vi "IMAQdx_AbsImage_Flea3_v4.7.vi"() -> ()   [LabVIEW 2013] (continued)
ODTpowHLat(DipPowHLat)\t0\tVimaging\t0\t0\t1\t0\t1\t1\t0\tbMOTpow(0.5)\tProbePow\t0\tXshimrMOT\tYshimrMOT\tZshimVar\tODTpowZ(DipPowZ)\tVimaging\t0\t0\tHimaging\t0\t0\t0\t0\t0\t0\t0\t0\t0\t0\t0\t0\t0\t0\trMOTdelta(-(rMOTstirDetI +stirWidthF/2))\tODTpowBlue(0)\tODTpowXY(DipPowCr)\tvarWaveP2\tProbePow2\tAmp688(depumpPow)\trMOTpow3\tODTpowX(DipPowX2)\tfreq\tHeatingAmp\t0\tSine\tDetuning\tsingleFreqDet +20\tDoppCoolDet-DoppCoolSweep\tdopCoolT*1000\tDetuning\tsingleFreqStirDet + 20\tsingleFreqStirDet + SFramp + SFramp2\tloadT*1000\tBlueBN\tBlueLaserProbeBN\tSSteckBN\tShortSteckDDS\tPixisPos(TOF)\tCycle Wait for Move\t0\t0\t0\t0\t0\t0\t0\t0\t0\t0\t0\t0\t0\t0\t0\t0\t0\t0\t0\t0\t0\t0\t0\t0\r\narm DIP FLEA\t\tRamp\t1\tcameraArmT\t0\t0\t0\t0\t0\t0\t0\t0\t0\t0\t0\t0\t0\t0\t0\t0\t0\t0\t0\t0\t0\t0\t0\t0\t0\t1\t1\t0\t0\t0\t1\t0\t0\tplus_zman\tminus_zman\tcompensation\trMOTcurrF\trMOTpow3\tcombAmplitude(combWidthF)\trMOTdelta(-(rMOTbroadDetuningF +combWidthF/2))\tODTpowHLat(DipPowHLat)\t0\tVimaging\t0\t0\t0\t0\t1\t0\t0\tbMOTpow(0.5)\tProbePow\t0\tXshimrMOT\tYshimrMOT\tZshimVar\tODTpowZ(DipPowZ3)\tVimaging\t0\t0\tHimaging\t0\t0\t0\t0\t0\t0\t0\t0\t0\t0\t0\t0\t0\t0\trMOTdelta(-(rMOTstirDetI +stirWidthF/2))\tODTpowBlue(0)\tODTpowXY(DipPowCrTOF)\tvarWaveP1\tProbePow2\tAmp688(depumpPow)\trMOTpow3\tODTpowX(DipPowXTOF)\tfreq\tHeatingAmp\t0\tSine\tDetuning\tsingleFreqDet +20\tDoppCoolDet-DoppCoolSweep\tdopCoolT*1000\tDetuning\tsingleFreqStirDet + 20\tsingleFreqStirDet + SFramp + SFramp2\tloadT*1000\tBlueBN\tBlueLaserProbeBN\tSSteckBN\tShortSteckDDS\tPixisPos(TOF)\tCycle Wait for Move\t0\t0\t0\t0\t0\t0\t0\t0\t0\t0\t0\t0\t0\t0\t0\t0\t0\t0\t0\t0\t0\t0\t0\t0\r\narm BEC FLEA\t\tRamp\t0\tcameraArmT\t1\t1\t1\t1\t1\t1\t0\t0\t0\t0\t0\t0\t0\t0\t0\t0\t0\t0\t0\t0\t0\t0\t0\t0\t0\t1\t1\t0\t0\t0\t1\t0\t0\tplus_zman\tminus_zman\tcompensation\trMOTcurrF\trMOTpow3\tcombAmplitude(combWidthF)\trMOTdelta(-(rMOTbroadDetuningF +combWidthF/2))\tODTpowHLat(DipPowHLat)\t0\tVimaging\t0\t0\t0\t0\t1\t0\t0\tbMOTpow(0.5)\tProbePow\t0\tXshimrMOT\tYshimrMOT\tZshimVar\tODTpowZ(DipPowZ3)\tVimaging\t0\t0\tHimaging\t0\t0\t0\t0\t0\t0\t0\t0\t0\t0\t0\t0\t0\t0\trMOTdelta(-(rMOTstirDetI +stirWidthF/2))\tODTpowBlue(BlueDipPow)\tExpFinal(tEvap1,ODTpowXY(DipPowCr2),ODTpowXY(DipPowCr3),tau)\tvarWaveP1\tProbePow2\tAmp688(depumpPow)\trMOTpow3\tExpFinal(tEvap1,ODTpowX(DipPowX2),ODTpowX(DipPowX3),tau)\tfreq\tHeatingAmp\t0\tSine\tDetuning\tsingleFreqDet +20\tDoppCoolDet-DoppCoolSweep\tdopCoolT*1000\tDetuning\tsingleFreqStirDet + 20\tsingleFreqStirDet + SFramp + SFramp2\tloadT*1000\tBlueBN\tBlueLaserProbeBN\tSSteckBN\tShortSteckDDS\tPixisPos(TOF)\tCycle Wait for Move\t0\t0\t0\t0\t0\t0\t0\t0\t0\t0\t0\t0\t0\t0\t0\t0\t0\t0\t0\t0\t0\t0\t0\t0\r\natom img\t\tRamp\t1\texposureT\t0\t0\t0\t0\t0\t0\t0\t0\t1\t0\t0\t0\t0\t1\t0\t0\t0\t0\t1\t0\t0\t0\t0\t0\t0\t1\t1\t0\t0\t0\t1\t0\t0\tplus_zman\tminus_zman\tcompensation\trMOTcurrF\trMOTpow3\tcombAmplitude(combWidthF)\trMOTdelta(-(rMOTbroadDetuningF +combWidthF/2))\tODTpowHLat(DipPowHLat)\t0\tVimaging\t0\t0\t0\t0\t0\t0\t0\tbMOTpow(0.5)\tProbePow\t0\tXshimrMOT\tYshimrMOT\tZshimVar\tODTpowZ(DipPowZ)\tVimaging\t0\t0\tHimaging\t0\t0\t0\t0\t0\t0\t0\t0\t0\t0\t0\t0\t0\t0\trMOTdelta(-(rMOTstirDetI +stirWidthF/2))\tODTpowBlue(BlueDipPow)\tODTpowXY(DipPowCr)\tvarWaveP1\tProbePow2\tAmp688(depumpPow)\trMOTpow3\tODTpowX(DipPowX)\tfreq\tHeatingAmp\t0\tSine\tDetuning\tsingleFreqDet +20\tDoppCoolDet-DoppCoolSweep\tdopCoolT*1000\tDetuning\tsingleFreqStirDet + 20\tsingleFreqStirDet + SFramp + SFramp2\tloadT*1000\tBlueBN\tBlueLaserProbeBN\tSSteckBN\tShortSteckDDS\tPixisPos(TOF)\tCycle Wait for Move\t0\t0\t0\t0\t0\t0\t0\t0\t0\t0\t0\t0\t0\t0\t0\t0\t0\t0\t0\t0\t0\t0\t0\t0\r\natom img\t\tRamp\t0\t2.8e-3\t0\t0\t0\t0\t0\t0\t0\t0\t0\t1\t0\t0\t0\t0\t0\t0\t0\t0\t0\t0\t0\t0\t0\t0\t0\t1\t1\t0\t0\t0\t1\t1\t0\tplus_zman\tminus_zman\tcompensation\trMOTcurrF\trMOTpow3\tcombAmplitude(combWidthF)\trMOTdelta(-(rMOTbroadDetuningF +combWidthF/2))\tODTpowHLat(DipPowHLat)\t0\tVimaging\t0\t0\t1\t0\t1\t1\t0\tbMOTpow(0.5)\tProbePow\t0\tXshimrMOT\tYshimrMOT\tZshimVar\tODTpowZ(DipPowZ)\tVimaging\t0\t0\tHimaging\t0\t0\t0\t0\t0\t0\t0\t0\t0\t0\t0\t0\t0\t0\trMOTdelta(-(rMOTstirDetI +stirWidthF/2))\tODTpowBlue(0)\tODTpowXY(DipPowCr)\tvarWaveP2\tProbePow2\tAmp688(depumpPow)\trMOTpow3\tODTpowX(DipPowX)\tfreq\tHeatingAmp\t0\tSine\tDetuning\tsingleFreqDet +20\tDoppCoolDet-DoppCoolSweep\tdopCoolT*1000\tDetuning\tsingleFreqStirDet + 20\tsingleFreqStirDet + SFramp + SFramp2\tloadT*1000\tBlueBN\tBlueLaserProbeBN\tSSteckBN\tShortSteckDDS\tPixisPos(TOF)\tCycle Wait for Move\t0\t0\t0\t0\t0\t0\t0\t0\t0\t0\t0\t0\t0\t0\t0\t0\t0\t0\t0\t0\t0\t0\t0\t0\r\ntransmit img\t\tRamp\t1\t.7\t0\t0\t0\t0\t0\t0\t0\t0\t0\t1\t0\t0\t0\t0\t0\t0\t0\t0\t0\t0\t0\t0\t0\t0\t0\t1\t1\t0\t0\t0\t1\t1\t0\tplus_zman\tminus_zman\tcompensation\trMOTcurrF\trMOTpow3\tcombAmplitude(combWidthF)\trMOTdelta(-(rMOTbroadDetuningF +combWidthF/2))\tODTpowHLat(DipPowHLat)\t0\tVimaging\t0\t0\t1\t0\t1\t1\t0\tbMOTpow(0.5)\tProbePow\t0\tXshimrMOT\tYshimrMOT\tZshimVar\tODTpowZ(DipPowZ)\tVimaging\t0\t0\t1\t0\t1\t0\t0\t0\t0\t0\t0\t0\t0\t0\t0\t0\t0\trMOTdelta(-(rMOTstirDetI +stirWidthF/2))\tODTpowBlue(0)\tODTpowXY(DipPowCr)\tvarWaveP2\tProbePow2\tAmp688(depumpPow)\trMOTpow3\tODTpowX(DipPowX)\tfreq\tHeatingAmp\t0\tSine\tDetuning\tsingleFreqDet +20\tDoppCoolDet-DoppCoolSweep\tdopCoolT*1000\tDetuning\tsingleFreqStirDet + 20\tsingleFreqStirDet + SFramp + SFramp2\tloadT*1000\tBlueBN\tBlueLaserProbeBN\tSSteckBN\tShortSteckDDS\tPixisPos(TOF)\tCycle Wait for Move\t0\t0\t0\t0\t0\t0\t0\t0\t0\t0\t0\t0\t0\t0\t0\t0\t0\t0\t0\t0\t0\t0\t0\t0\r\narm PIXIS\t\tRamp\t0\t.007\t0\t0\t0\t0\t0\t0\t0\t0\t0\t1\t1\t0\t0\t0\t1\t1\t0\t0\t0\t0\t0\t0\t0\t0\t0\t1\t1\t0\t0\t0\t1\t1\t0\tplus_zman\tminus_zman\tcompensation\trMOTcurrF\trMOTpow1\tcombAmplitude(combWidthF)\trMOTdelta(-(rMOTbroadDetuningF +combWidthF/2))\tODTpowHLat(DipPowHLat)\t0\tVimaging\t0\t0\t1\t0\t1\t1\t0\tbMOTpow(0.5)\tProbePow\t0\tXshimrMOT\tYshimrMOT\tZshimVar\tODTpowZ(DipPowZ)\tVimaging\t0\t0\t1\t0\t1\t0\t0\t0\t0\t0\t0\t0\t0\t0\t0\t0\t0\trMOTdelta(-(rMOTstirDetI +stirWidthF/2))\tODTpowBlue(0)\tODTpowXY(DipPowCr)\tvarWaveP2\tProbePow2\tAmp688(depumpPow)\trMOTpow1\tODTpowX(DipPowX)\tfreq\tHeatingAmp\t0\tSine\tDetuning\tsingleFreqDet +20\tDoppCoolDet-DoppCoolSweep\tdopCoolT*1000\tDetuning\tsingleFreqStirDet + 20\tsingleFreqStirDet + SFramp + SFramp2\tloadT*1000\tBlueBN\tBlueLaserProbeBN\tSSteckBN\tShortSteckDDS\tPixisPos(TOF)\tCycle Wait for Move\t0\t0\t0\t0\t0\t0\t0\t0\t0\t0\t0\t0\t0\t0\t0\t0\t0\t0\t0\t0\t0\t0\t0\t0\r\narm FLEA\t\tRamp\t1\tcameraArmT\t0\t0\t0\t0\t0\t0\t0\t0\t0\t1\t1\t0\t0\t0\t1\t1\t0\t0\t0\t0\t0\t0\t0\t0\t0\t1\t1\t0\t0\t0\t1\t0\t0\tplus_zman\tminus_zman\tcompensation\trMOTcurrF\trMOTpow1\tcombAmplitude(combWidthF)\trMOTdelta(-(rMOTbroadDetuningF +combWidthF/2))\tODTpowHLat(DipPowHLat)\t0\tVimaging\t0\t0\t0\t0\t1\t0\t0\tbMOTpow(0.5)\tProbePow\t0\tXshimrMOT\tYshimrMOT\tZshimVar\tODTpowZ(DipPowZ)\tVimaging\t0\t0\t0\t0\t1\t0\t0\t0\t0\t0\t0\t0\t0\t0\t0\t0\t0\trMOTdelta(-(rMOTstirDetI +stirWidthF/2))\tODTpowBlue(0)\tODTpowXY(DipPowCr)\tvarWaveP2\tProbePow2\tAmp688(depumpPow)\trMOTpow1\tODTpowX(DipPowX)\tfreq\tHeatingAmp\t0\tSine\tDetuning\tsingleFreqDet +20\tDoppCoolDet-DoppCoolSweep\tdopCoolT*1000\tDetuning\tsingleFreqStirDet + 20\tsingleFreqStirDet + SFramp + SFramp2\tloadT*1000\tBlueBN\tBlueLaserProbeBN\tSSteckBN\tShortSteckDDS\tPixisPos(TOF)\tCycle Wait for Move\t0\t0\t0\t0\t0\t0\t0\t0\t0\t0\t0\t0\t0\t0\t0\t0\t0\t0\t0\t0\t0\t0\t0\t0\r\nprobe img\t\tRamp\t1\texposureT\t0\t0\t0\t0\t0\t0\t0\t0\t1\t1\t1\t0\t0\t1\t1\t1\t0\t0\t0\t0\t0\t0\t0\t0\t0\t1\t1\t0\t0\t0\t1\t0\t0\tplus_zman\tminus_zman\tcompensation\trMOTcurrF\trMOTpow1\tcombAmplitude(combWidthF)\trMOTdelta(-(rMOTbroadDetuningF +combWidthF/2))\tODTpowHLat(DipPowHLat)\t0\tVimaging\t0\t0\t0\t0\t0\t0\t0\tbMOTpow(0.5)\tProbePow\t0\tXshimrMOT\tYshimrMOT\tZshimVar\tODTpowZ(DipPowZ)\tVimaging\t0\t0\t0\t0\t1\t0\t0\t0\t0\t0\t0\t0\t0\t0\t0\t0\t0\trMOTdelta(-(rMOTstirDetI +stirWidthF/2))\tODTpowBlue(0)\tODTpowXY(DipPowCr)\tvarWaveP2\tProbePow2\tAmp688(depumpPow)\trMOTpow1\tODTpowX(DipPowX)\tfreq\tHeatingAmp\t0\tSine\tDetuning\tsingleFreqDet +20\tDoppCoolDet-DoppCoolSweep\tdopCoolT*1000\tDetuning\tsingleFreqStirDet + 20\tsingleFreqStirDet + SFramp + SFramp2\tloadT*1000\tBlueBN\tBlueLaserProbeBN\tSSteckBN\tShortSteckDDS\tPixisPos(TOF)\tCycle Wait for Move\t0\t0\t0\t0\t0\t0\t0\t0\t0\t0\t0\t0\t0\t0\t0\t0\t0\t0\t0\t0\t0\t0\t0\t0\r\nprobe img\t\tRamp\t0\t2.8e-3\t0\t0\t0\t0\t0\t0\t0\t0\t0\t1\t1\t0\t0\t0\t1\t1\t0\t0\t0\t0\t0\t0\t0\t0\t0\t1\t1\t0\t0\t0\t1\t1\t0\tplus_zman\tminus_zman\tcompensation\trMOTcurrF\trMOTpow1\tcombAmplitude(combWidthF)\trMOTdelta(-(rMOTbroadDetuningF +combWidthF/2))\tODTpowHLat(DipPowHLat)\t0\tVimaging\t0\t0\t1\t0\t1\t1\t0\tbMOTpow(0.5)\tProbePow\t0\tXshimrMOT\tYshimrMOT\tZshimVar\tODTpowZ(DipPowZ)\tVimaging\t0\t0\t0\t0\t1\t0\t0\t0\t0\t0\t0\t0\t0\t0\t0\t0\t0\trMOTdelta(-(rMOTstirDetI +stirWidthF/2))\tODTpowBlue(0)\tODTpowXY(DipPowCr)\tvarWaveP2\tProbePow2\tAmp688(depumpPow)\trMOTpow1\tODTpowX(DipPowX)\tfreq\tHeatingAmp\t0\tSine\tDetuning\tsingleFreqDet +20\tDoppCoolDet-DoppCoolSweep\tdopCoolT*1000\tDetuning\tsingleFreqStirDet + 20\tsingleFreqStirDet + SFramp + SFramp2\tloadT*1000\tBlueBN\tBlueLaserProbeBN\tSSteckBN\tShortSteckDDS\tPixisPos(TOF)\tCycle Wait for Move\t0\t0\t0\t0\t0\t0\t0\t0\t0\t0\t0\t0\t0\t0\t0\t0\t0\t0\t0\t0\t0\t0\t0\t0\r\ntransmit img\t\tRamp\t1\t.600\t0\t0\t0\t0\t0\t0\t0\t0\t0\t1\t1\t0\t0\t0\t1\t1\t0\t0\t0\t0\t0\t0\t0\t0\t0\t1\t1\t0\t0\t0\t1\t1\t0\tplus_zman\tminus_zman\tcompensation\trMOTcurrF\trMOTpow1\tcombAmplitude(combWidthF)\trMOTdelta(-(rMOTbroadDetuningF +combWidthF/2))\tODTpowHLat(DipPowHLat)\t0\tVimaging\t0\t0\t1\t0\t1\t1\t0\tbMOTpow(0.5)\tProbePow\t0\tXshimrMOT\tYshimrMOT\tZshimVar\tODTpowZ(DipPowZ)\tVimaging\t0\t0\t0\t0\t1\t0\t0\t0\t0\t0\t0\t0\t0\t0\t0\t0\t0\trMOTdelta(-(rMOTstirDetI +stirWidthF/2))\tODTpowBlue(0)\tODTpowXY(DipPowCr)\tvarWaveP2\tProbePow2\tAmp688(depumpPow)\trMOTpow1\tODTpowX(DipPowX)\tfreq\tHeatingAmp\t0\tSine\tDetuning\tsingleFreqDet +20\tDoppCoolDet-DoppCoolSweep\tdopCoolT*1000\tDetuning\tsingleFreqStirDet + 20\tsingleFreqStirDet + SFramp + SFramp2\tloadT*1000\tBlueBN\tBlueLaserProbeBN\tSSteckBN\tShortSteckDDS\tPixisPos(TOF)\tCycle Wait for Move\t0\t0\t0\t0\t0\t0\t0\t0\t0\t0\t0\t0\t0\t0\t0\t0\t0\t0\t0\t0\t0\t0\t0\t0\r\ntransmit img\t\tRamp\t1\t.025\t0\t0\t0\t0\t0\t0\t0\t0\t0\t1\t1\t0\t0\t0\t1\t1\t0\t0\t0\t0\t0\t0\t0\t0\t0\t1\t1\t0\t0\t0\t1\t1\t0\tplus_zman\tminus_zman\tcompensation\trMOTcurrF\trMOTpow1\tcombAmplitude(combWidthF)\trMOTdelta(-(rMOTbroadDetuningF +combWidthF/2))\tODTpowHLat(DipPowHLat2)\t0\tVimaging\t0\t0\t1\t0\t1\t1\t0\tbMOTpow(0.5)\tProbePow\t0\tXshimrMOT\tYshimrMOT\tZshimVar\tODTpowZ(DipPowZ)\tVimaging\t0\t0\t0\t0\t1\t0\t0\t0\t0\t0\t0\t0\t0\t0\t0\t0\t0\trMOTdelta(-(rMOTstirDetI +stirWidthF/2))\tODTpowBlue(.05)\tODTpowXY(DipPowCr)\tvarWaveP2\tProbePow2\tAmp688(depumpPow)\trMOTpow1\tODTpowX(DipPowX)\tfreq\tHeatingAmp\t0\tSine\tDetuning\tsingleFreqDet +20\tDoppCoolDet-DoppCoolSweep\tdopCoolT*1000\tDetuning\tsingleFreqStirDet + 20\tsingleFreqStirDet + SFramp + SFramp2\tloadT*1000\tBlueBN\tBlueLaserProbeBN\tSSteckBN\tShortSteckDDS\tPixisPos(TOF)\tCycle Wait for Move\t0\t0\t0\t0\t0\t0\t0\t0\t0\t0\t0\t0\t0\t0\t0\t0\t0\t0\t0\t0\t0\t0\t0\t0\r\narm PIXIS\t\tRamp\t0\t.007\t0\t0\t0\t0\t0\t0\t0\t0\t0\t1\t1\t0\t0\t0\t1\t1\t0\t0\t0\t0\t0\t0\t0\t0\t0\t1\t1\t0\t0\t0\t1\t0\t0\tplus_zman\tminus_zman\tcompensation\trMOTcurrF\trMOTpow1\tcombAmplitude(combWidthF)\trMOTdelta(-(rMOTbroadDetuningF +combWidthF/2))\tODTpowHLat(DipPowHLat2)\t0\tVimaging\t0\t0\t0\t0\t1\t1\t0\tbMOTpow(0.5)\tProbePow\t0\tXshimrMOT\tYshimrMOT\tZshimVar\tODTpowZ(DipPowZ)\tVimaging\t0\t0\t0\t0\t1\t0\t0\t0\t0\t0\t0\t0\t0\t0\t0\t0\t0\trMOTdelta(-(rMOTstirDetI +stirWidthF/2))\tODTpowBlue(0)\tODTpowXY(DipPowCr)\tvarWaveP2\tProbePow2\tAmp688(depumpPow)\trMOTpow1\tODTpowX(DipPowX)\tfreq\tHeatingAmp\t0\tSine\tDetuning\tsingleFreqDet +20\tDoppCoolDet-DoppCoolSweep\tdopCoolT*1000\tDetuning\tsingleFreqStirDet + 20\tsingleFreqStirDet + SFramp + SFramp2\tloadT*1000\tBlueBN\tBlueLaserProbeBN\tSSteckBN\tShortSteckDDS\tPixisPos(TOF)\tCycle Wait for Move\t0\t0\t0\t0\t0\t0\t0\t0\t0\t0\t0\t0\t0\t0\t0\t0\t0\t0\t0\t0\t0\t0\t0\t0\r\narm FLEA\t\tRamp\t1\tcameraArmT\t0\t0\t0\t0\t0\t0\t0\t0\t0\t1\t1\t0\t0\t0\t1\t1\t0\t0\t0\t0\t0\t0\t0\t0\t0\t1\t1\t0\t0\t0\t1\t0\t0\tplus_zman\tminus_zman\tcompensation\trMOTcurrF\trMOTpow1\tcombAmplitude(combWidthF)\trMOTdelta(-(rMOTbroadDetuningF +combWidthF/2))\tODTpowHLat(DipPowHLat2)\t0\tVimaging\t0\t0\t0\t0\t1\t0\t0\tbMOTpow(0.5)\tProbePow\t0\tXshimrMOT\tYshimrMOT\tZshimVar\tODTpowZ(DipPowZ)\tVimaging\t0\t0\t0\t0\t1\t0\t0\t0\t0\t0\t0\t0\t0\t0\t0\t0\t0\trMOTdelta(-(rMOTstirDetI +stirWidthF/2))\tODTpowBlue(.05)\tODTpowXY(DipPowCr)\tvarWaveP2\tProbePow2\tAmp688(depumpPow)\trMOTpow1\tODTpowX(DipPowX)\tfreq\tHeatingAmp\t0\tSine\tDetuning\tsingleFreqDet +20\tDoppCoolDet-DoppCoolSweep\tdopCoolT*1000\tDetuning\tsingleFreqStirDet + 20\tsingleFreqStirDet + SFramp + SFramp2\tloadT*1000\tBlueBN\tBlueLaserProbeBN\tSSteckBN\tShortSteckDDS\tPixisPos(TOF)\tCycle Wait for Move\t0\t0\t0\t0\t0\t0\t0\t0\t0\t0\t0\t0\t0\t0\t0\t0\t0\t0\t0\t0\t0\t0\t0\t0\r\nbg img\t\tRamp\t1\texposureT\t0\t0\t0\t0\t0\t0\t0\t0\t0\t1\t1\t0\t0\t0\t1\t1\t0\t0\t0\t0\t0\t0\t0\t0\t0\t1\t1\t0\t0\t0\t1\t0\t0\tplus_zman\tminus_zman\tcompensation\trMOTcurrF\trMOTpow1\tcombAmplitude(combWidthF)\trMOTdelta(-(rMOTbroadDetuningF +combWidthF/2))\tODTpowHLat(DipPowHLat2)\t0\tVimaging\t0\t0\t0\t0\t0\t0\t0\tbMOTpow(0.5)\tProbePow\t0\tXshimrMOT\tYshimrMOT\tZshimVar\tODTpowZ(DipPowZ)\tVimaging\t0\t0\t0\t0\t1\t0\t0\t0\t0\t0\t0\t0\t0\t0\t0\t0\t0\trMOTdelta(-(rMOTstirDetI +stirWidthF/2))\tODTpowBlue(.05)\tODTpowXY(DipPowCr)\tvarWaveP2\tProbePow2\tAmp688(depumpPow)\trMOTpow1\tODTpowX(DipPowX)\tfreq\tHeatingAmp\t0\tSine\tDetuning\tsingleFreqDet +20\tDoppCoolDet-DoppCoolSweep\tdopCoolT*1000\tDetuning\tsingleFreqStirDet + 20\tsingleFreqStirDet + SFramp + SFramp2\tloadT*1000\tBlueBN\tBlueLaserProbeBN\tSSteckBN\tShortSteckDDS\tPixisPos(TOF)\tCycle Wait for Move\t0\t0\t0\t0\t0\t0\t0\t0\t0\t0\t0\t0\t0\t0\t0\t0\t0\t0\t0\t0\t0\t0\t0\t0\r\nbg img\t\tRamp\t0\t1e-4\t0\t0\t0\t0\t0\t0\t0\t0\t0\t1\t1\t0\t0\t0\t1\t1\t0\t0\t0\t0\t0\t0\t0\t0\t0\t1\t1\t0\t0\t0\t1\t1\t0\tplus_zman\tminus_zman\tcompensation\trMOTcurrF\trMOTpow1\tcombAmplitude(combWidthF)\trMOTdelta(-(rMOTbroadDetuningF +combWidthF/2))\tODTpowHLat(DipPowHLat)\t0\tVimaging\t0\t0\t1\t0\t1\t1\t0\tbMOTpow(0.5)\tProbePow\t0\tXshimrMOT\tYshimrMOT\tZshimVar\tODTpowZ(DipPowZ)\tVimaging\t0\t0\t0\t0\t1\t0\t0\t0\t0\t0\t0\t0\t0\t0\t0\t0\t0\trMOTdelta(-(rMOTstirDetI +stirWidthF/2))\tODTpowBlue(0)\tODTpowXY(DipPowCr)\tvarWaveP2\tProbePow2\tAmp688(depumpPow)\trMOTpow1\tODTpowX(DipPowX)\tfreq\tHeatingAmp\t0\tSine\tDetuning\tsingleFreqDet +20\tDoppCoolDet-DoppCoolSweep\tdopCoolT*1000\tDetuning\tsingleFreqStirDet + 20\tsingleFreqStirDet + SFramp + SFramp2\tloadT*1000\tBlueBN\tBlueLaserProbeBN\tSSteckBN\tShortSteckDDS\tPixisPos(TOF)\tCycle Wait for Move\t0\t0\t0\t0\t0\t0\t0\t0\t0\t0\t0\t0\t0\t0\t0\t0\t0\t0\t0\t0\t0\t0\t0\t0\r\ntransmit img\t\tRamp\t1\t.625\t0\t0\t0\t0\t0\t0\t0\t1\t0\t1\t1\t0\t0\t0\t1\t1\t0\t0\t0\t0\t0\t0\t0\t0\t0\t1\t1\t0\t0\t0\t1\t1\t0\tplus_zman\tminus_zman\tcompensation\trMOTcurrF\trMOTpow1\tcombAmplitude(combWidthF)\trMOTdelta(-(rMOTbroadDetuningF +combWidthF/2))\tODTpowHLat(DipPowHLat)\t0\tVimaging\t0\t0\t1\t0\t1\t1\t0\tbMOTpow(0.5)\tProbePow\t0\tXshimrMOT\tYshimrMOT\tZshimVar\tODTpowZ(DipPowZ)\tVimaging\t0\t0\t0\t0\t1\t0\t0\t0\t0\t0\t0\t0\t0\t0\t0\t0\t0\trMOTdelta(-(rMOTstirDetI +stirWidthF/2))\tODTpowBlue(0)\tODTpowXY(DipPowCr)\tvarWaveP2\tProbePow2\tAmp688(depumpPow)\trMOTpow1\tODTpowX(DipPowX)\tfreq\tHeatingAmp\t0\tSine\tDetuning\tsingleFreqDet +20\tDoppCoolDet-DoppCoolSweep\tdopCoolT*1000\tDetuning\tsingleFreqStirDet + 20\tsingleFreqStirDet + SFramp + SFramp2\tloadT*1000\tBlueBN\tBlueLaserProbeBN\tSSteckBN\tShortSteckDDS\tPixisPos(TOF)\tCycle Wait for Move\t0\t0\t0\t0\t0\t0\t0\t0\t0\t0\t0\t0\t0\t0\t0\t0\t0\t0\t0\t0\t0\t0\t0\t0\r\nalignment\t\tRamp\t1\t.1\t1\t1\t1\t1\t1\t1\t1\t0\t1\t0\t1\t0\t1\t1\t1\t1\t0\t0\t0\t0\t0\t0\t0\t0\t1m\t1\t1\t0\t1\t0\t0\t1\t1\tplus_zman\tminus_zman\tcompensation\tMOTcurrent\trMOTpow1\tcombAmplitude(combWidthI)\trMOTdelta(-(rMOTbroadDetuningI +combWidthI/2))\tODTpowHLat(DipPowHLat2)\t1\t0\t1\t1\t1\t1\t1\t1\t0\tbMOTpow(MOTPow)\tProbePow\t0\tXshim\tYshim\tZshim\tODTpowZ(DipPowZ3)\t0\t1\t1\t0\t1\t1\t0\t1\t0\t0\t0\t0\t0\t0\t0\t0\t0\t0\trMOTdelta(-(rMOTstirDetI +stirWidthI/2))\tODTpowBlue(0.05)\tExpFinal(tEvap1,ODTpowXY(DipPowCr2),ODTpowXY(DipPowCr3),tau)\tvarWaveP2\tProbePow2\tAmp688(depumpPow)\trMOTpow3\tExpFinal(tEvap1,ODTpowX(DipPowX2),ODTpowX(DipPowX3),tau)\tfreq\tHeatingAmp\t0\tSine\tDetuning\tsingleFreqDet +20\tDoppCoolDet-DoppCoolSweep\tdopCoolT*1000\tDetuning\tsingleFreqStirDet + 20\tsingleFreqStirDet + SFramp + SFramp2\tloadT*1000\tBlueBN\tBlueLaserBeatnote\tSSteckBN\tShortSteckDDS\tPixisPos(TOF)\tCycle Wait for Move\t0\t0\t0\t0\t0\t0\t0\t0\t0\t0\t0\t0\t0\t0\t0\t0\t0\t0\t0\t0\t0\t0\t0\t0\r\n\r\n\r\n"
  in  "Flea Wave Name":string="Test_Img"
  in  "Save files to archive?":bool
  out "Timeout":bool
  out "Trigger Overrun":bool
  in  "Source of File Data":refnum<k21>="\\\\Control\\VariableLibrary\\Instruction String"
  in  "Timeout (ms)":u32=20000
  in  "Gain":dbl
  in  "Shutter speed":dbl=30000.0
  in  "PIXIS Magnification":dbl=5.48
  in  "PIXIS Image direction":enum16{"XY", "XZ"}(ring)
  in  "PIXIS Imaging technique":enum16{"Absorption", "Fluorescence", "RawImage"}(ring)
  in  "SPE File Path":path=path "C:/Users/Lab/Documents/LightField/LabviewTemp.spe"
  in  "Send PIXIS data to Igor?":bool
  in  "PIXIS File Parameters":T1={"Data Root"=path "I:/Data", "Index"=3939, "Instrument"="PIXIS"} {"Index" format="%04d"}
  in  "Source of Wavemeter Data":refnum<k21>="\\\\WS7PC\\VariableLibrary\\Frequency"
  in  "Accept wavelength from remote system":bool=TRUE
  in  "Flea Raw image to view":u16(ring) items=["Clear", "Absorbtion", "Probe", "Background"]
  in  "Update Graphics":bool=TRUE
  out "Flea Raw Image":u16[][](graph)
  out "Flea Processed Image":sgl[][](graph)
  out "PIXIS Processed Image":sgl[][](graph)
  out "PIXIS Raw Image":u16[][](graph)
  in  "PIXIS Raw image to view":u16(ring)=1 items=["Clear", "Absorbtion", "Probe", "Background"]
  out "Camera Error":errorcluster
  out "DDE Error":errorcluster={"status"=TRUE, "code"=14012, "source"="DDE Execute: DMLERR_NOTPROCESSED"}
  out "Status Array":T4(array[cluster])=[{"AcquisitionInProgress"=FALSE, "BufferCount"=0, "LastBufferNumber"=4294967292, "LostBufferCount"=0}, {"AcquisitionInProgress"=TRUE, "BufferCount"=0, "LastBufferNumber"=4294967292, "LostBufferCount"=0}, {"AcquisitionInProgress"=TRUE, "BufferCount"=0, "LastBufferNumber"=4294967292, "LostBufferCount"=0}, {"AcquisitionInProgress"=TRUE, "BufferCount"=1, "LastBufferNumber"=0, "LostBufferCount"=0}, {"AcquisitionInProgress"=TRUE, "BufferCount"=2, "LastBufferNumber"=1, "LostBufferCount"=0}, {"AcquisitionInProgress"=TRUE, "BufferCount"=3, "LastBufferNumber"=2, "LostBufferCount"=0}, {"AcquisitionInProgress"=TRUE, "BufferCount"=4, "LastBufferNumber"=3, "LostBufferCount"=0}]
  in  "SPE Load Error In":errorcluster
  out "DataBlock Info":T5={"frame count"=4, "frame size"=2097152, "frame stride"=2097152, "N ROI"=1, "ROI widths"=[1024], "ROI heights"=[1024], "ROI sizes"=[2097152], "ROI strides"=[2097152]}
  out "DS Error":errorcluster
  out "XML Parse Errors":string
  out "Data Array Size":i32=1
  out "SPE Load Error Out":errorcluster
  out "Flea Path":path=path "I:/Data/FL3_32S2Mtemp.ibw"
  out "PIXIS Path":path=path "I:/Data/PIXIStemp.ibw"
  out "PIXIS Images":u16[][][](array[numeric])
  out "Flea Images":u16[][][](array[numeric])
  out "Buffer Number":u32=3
  out "Flea Frames":i32=3
  out "Flea Loop":i32=31
  # "Image Acquisition v4.6 (FOR USB3 CAMERAS ONLY!!!)"
  # "Experimental Parameters"
  # "These are only get set on 1st run.\nUse a Gain of 0, Shutter Speed not used"
  # "In both techniques 3 images\nare aquired, but in Fluorescense\nthe 3rd is discarded"
  # "Sr: .663  is XZ a\n     .898 is XZ b\n      5.48 is XY"
  # "Obsolete: (now done with network variables)\nWhen paramaters are accepted from a remote system a DataSockets server\nmust be running on this machine (in start menu in National Instruments folder)"
  # "Camera configuration"
  # "File configuration"
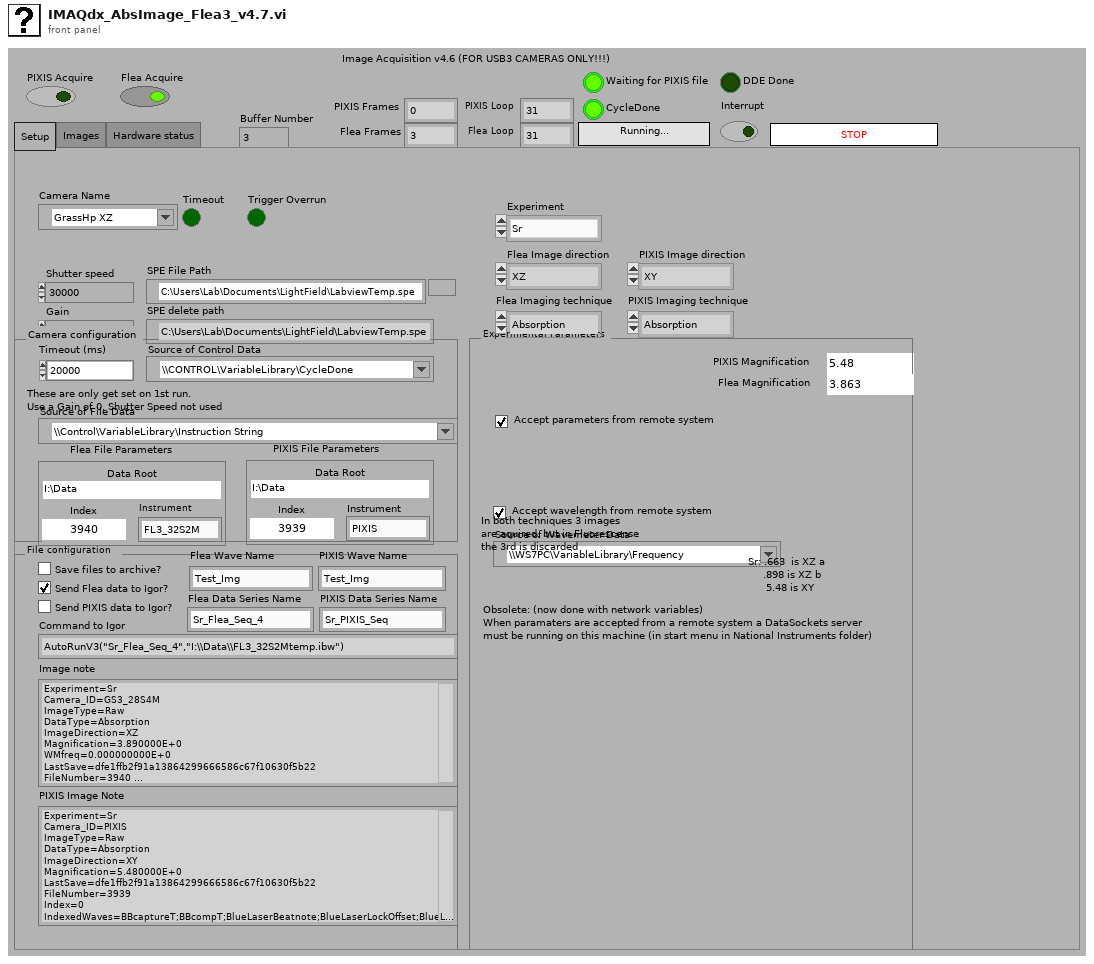
[diagram p1: front panel]
types:
  T1 = typedef "FileName_Cluster.ctl" = cluster{"Data Root":path, "Index":u32, "Instrument":string}
  T2 = typedef "IMAQdx.ctl" = refnum<k21>
  T3 = enum16{"Rubidium I", "Rubidium II", "RbLi", "RbYb", "Sr"}
  T4 = cluster{"AcquisitionInProgress":bool, "BufferCount":u32, "LastBufferNumber":u32, "LostBufferCount":u32}[]
  T5 = cluster{"frame count":i64, "frame size":i64, "frame stride":i64, "N ROI":i64, "ROI widths":i64[], "ROI heights":i64[], "ROI sizes":i64[], "ROI strides":i64[]}
  T6 = typedef "NI_Vision_Acquisition_Software.lvlib/IMAQdx Acquisition Mode.ctl" = enum32{"One Shot", "Continuous"}
  T7 = typedef "Image Type" = u32
  T8 = typedef "IMAQ Image.ctl" = refnum<image>
  T9 = cluster{"AcquisitionInProgress":bool, "BufferCount":u32, "LastBufferNumber":u32, "LostBufferCount":u32}
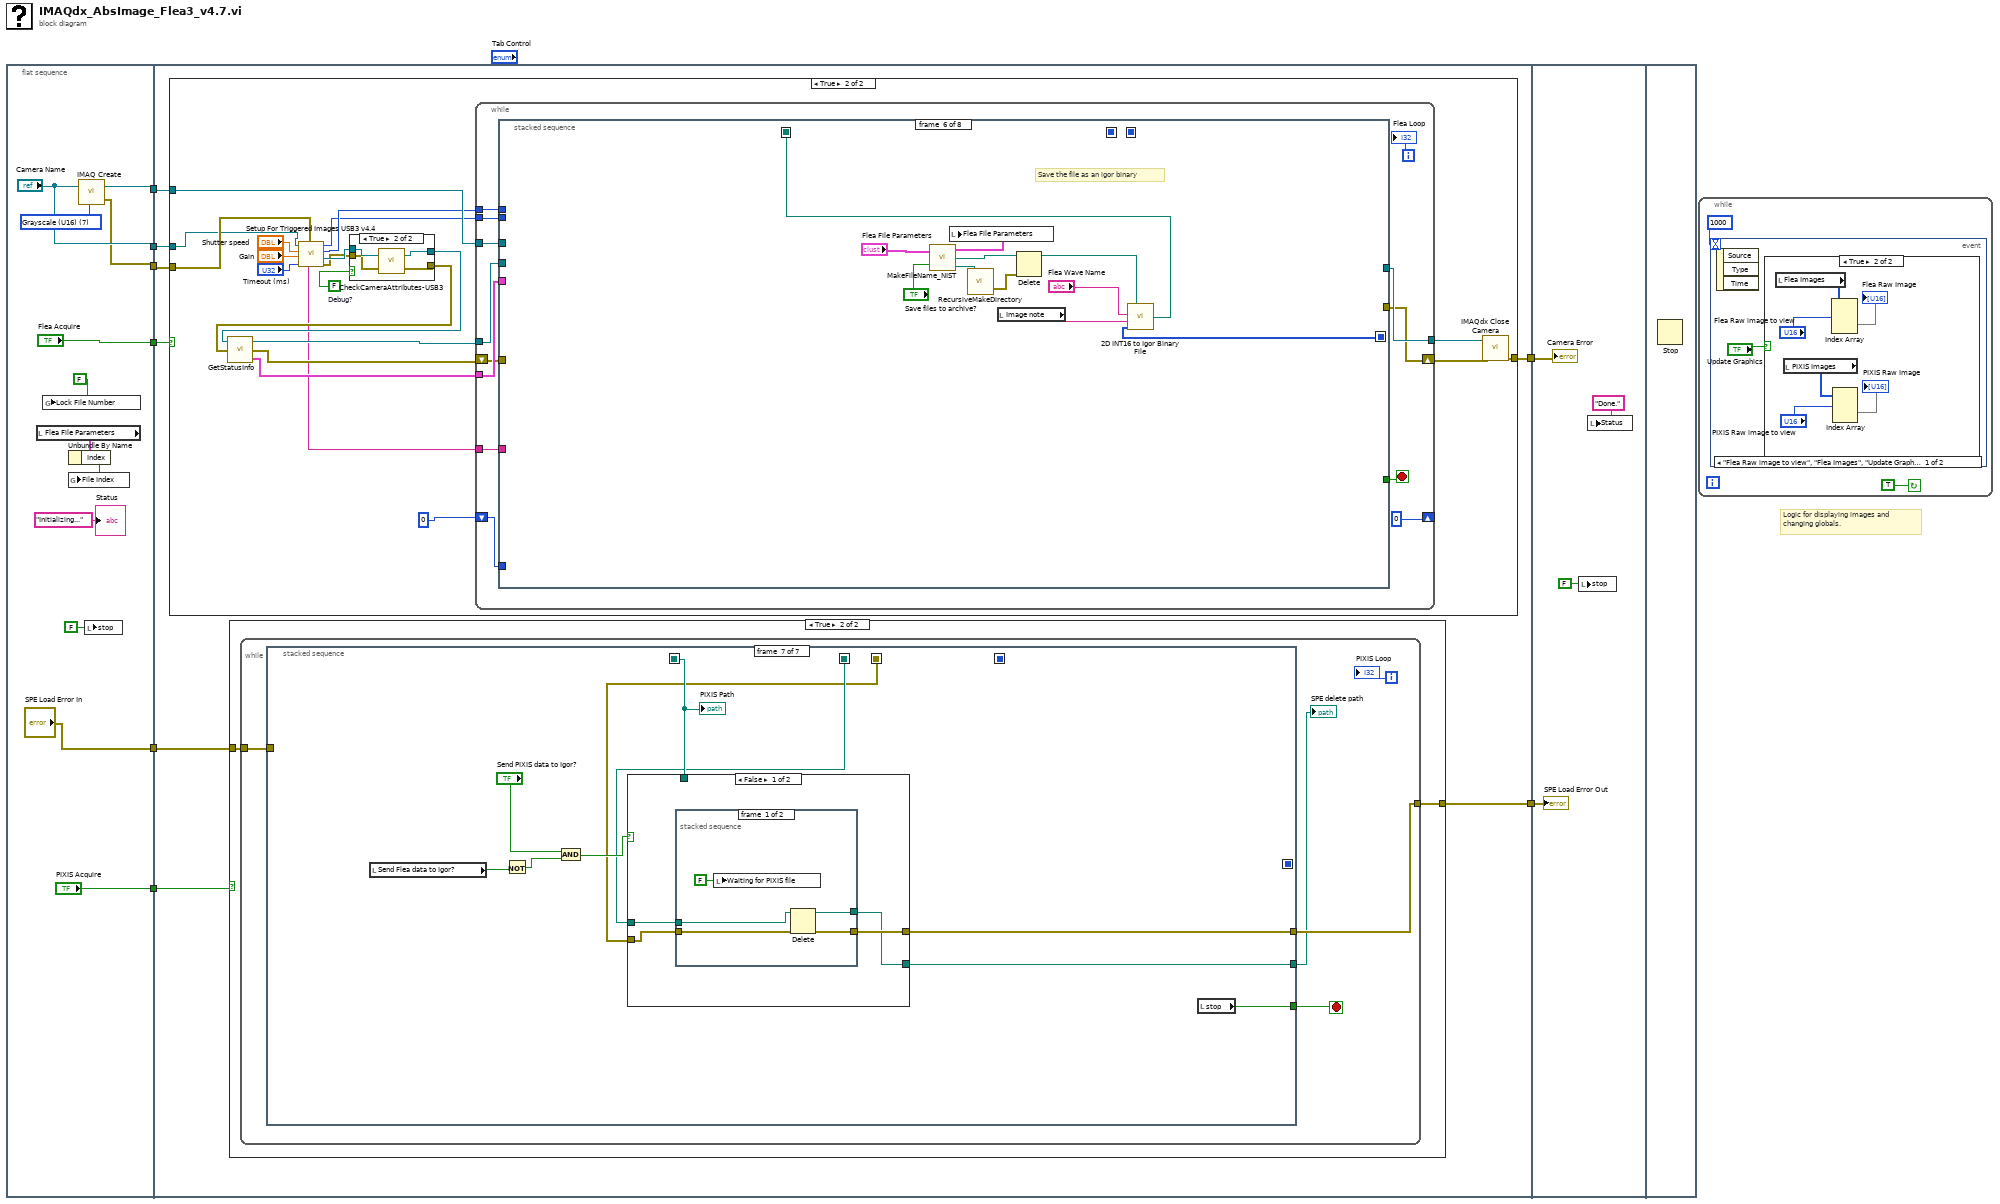
[diagram p0: block diagram]
diagram:
  # "Logic for displaying images and\nchanging globals."
  n1 = flat-sequence {
    tunnel: [w16] -> w8
    tunnel: ["Camera Name"] -> w7
    tunnel: [w14] -> w6
    tunnel: ["SPE Load Error In"] -> w5
    tunnel: ["PIXIS Acquire"] -> w3
    tunnel: ["Flea Acquire"] -> w1
    tunnel: w7 -> [w28]
    tunnel: w8 -> [w26]
    tunnel: w6 -> [w27]
    tunnel: w5 -> [w25]
    tunnel: [w24] -> w4
    tunnel: w3 -> [w23]
    tunnel: [w22] -> w2
    tunnel: w1 -> [w21]
    tunnel: w4 -> [w473]
    tunnel: w2 -> [w472]
    frame #0 {
      w13 = T7 7 items=["Grayscale (U8)", "Grayscale (I16)", "Grayscale (SGL)", "Complex (CSG)", "RGB (U32)", "HSL (U32)", "RGB (U64)", "Grayscale (U16)"] ("Image Type")
      n2 = local read "Flea File Parameters"() -> (w17:T1)
      n3 = global write "FileInfo_Global.vi" "Lock File Number"(FALSE) -> ()
      n4 = Unbundle By Name(w17) -> ("Index"=w18:u32)
      n5 = global write "FileInfo_Global.vi" "File Index"(w18) -> ()
      n6 = call "IMAQ Create"("Image Name"="Camera Name", "Image Type"=w13) -> ("New Image"=w16:T8, "error out"=w14:errorcluster)  [unwired: 2 in, 1 out]
      n7 = local write "stop"(FALSE ("stop")) -> ()
      "Status" <- "Initializing..."
    }
    frame #1 {
      n8 = case shown="True" w21 {
        tunnel: w28 -> [_ w34]
        tunnel: w27 -> [w29 w35]
        tunnel: w26 -> [_ w47]
        tunnel: [w29 w44] -> w22
        frame False {
        }
        frame True {
          w50 = FALSE  # Debug?
          n9 = call "Setup For Triggered Images USB3 v4.4.vi"("error in"=w35, "Timeout"="Timeout (ms)", "Gain"="Gain", "Shutter speed"="Shutter speed", "Camera Name"=w34) -> ("Error out"=w38:errorcluster, "Session Out"=w39:T2, "Height"=w37:u32, "Width"=w36:u32, "DeviceID"=w30:string)
          n10 = case shown="True" w50 {
            tunnel: [w51 w55] -> w49
            tunnel: [w52 w54] -> w48
            tunnel: w39 -> [w51 w56]
            tunnel: w38 -> [w52 w53]
            frame False {
            }
            frame True {
              n11 = call "CheckCameraAttributes-USB3.vi"("error in"=w53, "Camera Name"=w56) -> ("error out"=w54:errorcluster, "Session Out"=w55:T2)
            }
          }
          n12 = call "GetStatusInfo.vi"("error in"=w48, "Camera In"=w49) -> ("Status Info"=w46:T9, "error out"=w43:errorcluster, "Camera Out"=w42:T2)  [unwired: 1 in]
          n13 = while {
            tunnel: w42 -> [w67]
            tunnel: w47 -> [w66]
            tunnel: w37 -> [w65]
            tunnel: w36 -> [w64]
            tunnel: w46 -> [w63]
            tunnel: [w62] -> w41
            shift-right: [0] -> _
            shift-left: 0 -> [w61]
            shift-right: [w58] -> w40
            shift-left: w43 -> [w59]
            tunnel: w30 -> [w57]
            i -> [w69]
            stop <- w68 stop-if-true
            n14 = stacked-sequence {
              seq-local: [_ _ _ w184 _ _ _ _] -> [_ _ _ _ _ w258 _ _]
              seq-local: [_ _ _ _ _ w254 _ _] -> [_ _ _ _ _ _ _ w268]
              seq-local: [_ w89 _ _ _ _ _ _] -> [_ _ w158 _ _ _ _ _]
              seq-local: [_ _ w157 _ _ _ _ _] -> [_ _ _ w175 _ _ _ _]
              tunnel: [_ _ _ _ _ _ _ "stop"] -> w68
              tunnel: w67 -> [_ w81 _ _ _ _ _ _]
              tunnel: w66 -> [_ w97 _ _ _ _ _ _]
              tunnel: w65 -> [_ w96 _ _ _ _ _ _]
              tunnel: w64 -> [_ w95 _ _ _ _ _ _]
              tunnel: w63 -> [_ w93 _ _ _ _ _ _]
              tunnel: [_ w76 _ _ _ _ _ _] -> w62
              tunnel: [_ w75 _ _ _ _ _ _] -> w58
              tunnel: w61 -> [_ w92 _ _ _ _ _ _]
              tunnel: w59 -> [_ w84 _ _ _ _ _ _]
              tunnel: w57 -> [_ _ _ _ w205 _ _ _]
              frame #0 {
                n15 = local read "Send Flea data to Igor?"() -> (w70:bool)
                n16 = local write "Flea Frames"(0) -> ()
                n17 = local write "Status"("Running...") -> ()
                n18 = case shown="False" w70 {
                  frame False {
                    n19 = local write "DDE Done"(TRUE ("DDE Done")) -> ()
                  }
                  frame True {
                    "DDE Done" <- FALSE
                  }
                }
              }
              frame #1 {
                n20 = call <vilib>:"IMAQdx Configure Acquisition.vi"("error in"=w84, "Number of Buffers"=u32 5, "Continuous?"=IMAQdx_Acquisition_Mode."Continuous", "Session In"=w81) -> ("error out"=w83:errorcluster, "Session Out"=w82:T2)  [unwired: 6 in]
                n21 = call <vilib>:"IMAQdx Start Acquisition.vi"("error in"=w83, "Session In"=w82) -> ("error out"=w85:errorcluster, "Session Out"=w88:T2)  [unwired: 8 out]
                n22 = local write "Camera Error"(w85) -> ()
                n23 = Build Array(w93) -> (w94:T4)
                n24 = Initialize Array(u16 0, 4, w96, w95) -> (w99:u16[][][])
                n25 = while {
                  shift-right: [w111] -> _
                  shift-left: _ -> [w135]
                  tunnel: [w119] -> w87
                  tunnel: [w116] -> w91
                  shift-right: [w126] -> _
                  shift-left: w92 -> [w113]
                  shift-right: [w131] -> w89
                  shift-left: w99 -> [w132]
                  shift-right: [w114] -> w98
                  shift-left: w94 -> [w115]
                  tunnel: w88 -> [w110]
                  tunnel: w97 -> [w109]
                  tunnel: w85 -> [w108]
                  stop <- w122 continue-if-true
                  # "(Timeout code = -1074364414, IMAQ)\n(Timeout code = -1074360293, IMAQdx)\nDon't timeout waiting for first\nimage."
                  n26 = call <vilib>:"IMAQdx Grab.vi"("error in"=w108, "Wait for Next Buffer? (Yes)"=TRUE, "Image In"=w109, "Session In"=w110) -> ("error out"=w130:errorcluster, "Buffer Number Out"=w111:u32, "Image Out"=w125:T8, "Session Out"=w118:T2)  [unwired: 4 out]
                  "Buffer Number" <- w111
                  n27 = Unbundle By Name(w130) -> ("code"=w139:i32)
                  n28 = call "IMAQ ImageToArray"("Image"=w125) -> ("Image Pixels (U16)"=w124:u16[][])  [unwired: 2 in, 5 out]
                  n29 = case shown="0, Default" w139 {
                    tunnel: w130 -> [w144 w148]
                    tunnel: [w144 w147] -> w117
                    tunnel: [FALSE TRUE] -> w140
                    tunnel: w113 -> [w142 w146]
                    tunnel: [w141 w145] -> w126
                    frame 0, Default {
                      n30 = Increment(x=w142) -> (x+1=w141:i32)
                    }
                    frame -1074364414, -1074360293 {
                      n31 = case shown="0" w146 {
                        tunnel: [w150 w156] -> w147
                        tunnel: w148 -> [w152 w156]
                        tunnel: w146 -> [w151 w155]
                        tunnel: [w151 w154] -> w145
                        frame 0 {
                          n32 = Bundle By Name(cluster=w152, "status"=FALSE) -> (w150:errorcluster)
                        }
                        frame 1, Default {
                          n33 = Increment(x=w155) -> (x+1=w154:i32)
                        }
                      }
                    }